vi "FlexMag - 24-03-2023.vi"() -> ()   [LabVIEW 2018] (continued)
                                n18129 = local read "abort ch1"() -> (w22192:bool)
                                n18130 = Wait Until Next ms Multiple(millisecond multiple=u32 200) -> ()  [unwired: 1 out]
                                n18131 = Not(x=w22194) -> (.not. x?=w22193:bool)
                                n18132 = Compound Arithmetic op=OR(w22190, w22192, w22193) -> (w22191:bool)
                                }
                              }
                            }
                          }
                        }
                      }
                      frame True {
                      }
                    }
                  }
                }
              }
              frame #16 {
                n18133 = local read "ch1 shutdown alg"() -> (w22200:bool)
                n18134 = case shown="True" w22200 {
                  frame False {
                  }
                  frame True {
                    n18135 = local read "abort ch1"() -> (w22201:bool)
                    n18136 = case shown="False" w22201 {
                      frame False {
                        n18137 = local read "ch1 vent?"() -> (w22202:bool)
                        n18138 = case shown="False" w22202 {
                          frame False {
                            n18139 = local write "ch1 sd pcgv close led"(TRUE ("ch1 sd cc close led")) -> ()
                            n18140 = Wait (ms)(milliseconds to wait=u32 1000) -> ()  [unwired: 1 out]
                          }
                          frame True {
                            n18141 = local write "ch1 sd pcgv open led"(TRUE ("ch1 sd cc close led")) -> ()
                            n18142 = Wait (ms)(milliseconds to wait=u32 1000) -> ()  [unwired: 1 out]
                          }
                        }
                      }
                      frame True {
                      }
                    }
                  }
                }
              }
              frame #17 {
                n18143 = local read "ch1 shutdown alg"() -> (w22207:bool)
                n18144 = case shown="True" w22207 {
                  frame False {
                  }
                  frame True {
                    n18145 = local read "abort ch1"() -> (w22208:bool)
                    n18146 = case shown="False" w22208 {
                      frame False {
                        n18147 = local read "ch1 vent?"() -> (w22209:bool)
                        n18148 = case shown="True" w22209 {
                          frame False {
                            n18149 = while {
                              i -> [w22216]
                              stop <- w22212 stop-if-true
                              n18150 = Greater Or Equal?(x=w22216, y=200) -> (x >= y?=w22218:bool)
                              n18151 = case shown="True" w22218 {
                                frame False {
                                }
                                frame True {
                                n18152 = local write "ch1 shutdown error"(TRUE ("ch1 pumpdown error")) -> ()
                                n18153 = local write "Warning Message"("CH1 ShutDown process  is canceled !\nCH1 Trns BP Left couldn't be closed" ("Warning Message")) -> ()
                                }
                              }
                              n18154 = local read "CH1_Trns_BP_Left_DI"() -> (w22211:bool)
                              n18155 = case shown="True" w22211 {
                                tunnel: [TRUE FALSE] -> w22210
                                frame False {
                                }
                                frame True {
                                n18156 = Wait Until Next ms Multiple(millisecond multiple=u32 200) -> ()  [unwired: 1 out]
                                n18157 = local write "CH1_Trns_BP_Left_DO"(FALSE ("CH1_WFC_DO")) -> ()
                                }
                              }
                              n18158 = local read "abort ch1"() -> (w22213:bool)
                              n18159 = local read "ch1 shutdown alg"() -> (w22215:bool)
                              n18160 = Not(x=w22215) -> (.not. x?=w22214:bool)
                              n18161 = Compound Arithmetic op=OR(w22210, w22213, w22214) -> (w22212:bool)
                            }
                          }
                          frame True {
                            n18162 = local read "ch1_2 vacuum level"() -> (w22226:string)
                            n18163 = Equal?(x=w22226, y="VACUUM") -> (x = y?=w22227:bool)
                            n18164 = case shown="True" w22227 {
                              frame False {
                              }
                              frame True {
                                n18165 = while {
                                i -> [w22234]
                                stop <- w22230 stop-if-true
                                n18166 = Greater Or Equal?(x=w22234, y=100) -> (x >= y?=w22236:bool)
                                n18167 = case shown="True" w22236 {
                                frame False {
                                }
                                frame True {
                                n18168 = local write "ch1 shutdown error"(TRUE ("ch1 pumpdown error")) -> ()
                                n18169 = local write "Warning Message"("CH1 ShutDown process  is canceled !\nCH1 Trns BP Left couldn't be opened" ("Warning Message")) -> ()
                                }
                                }
                                n18170 = local read "CH1_Trns_BP_Left_DI"() -> (w22229:bool)
                                n18171 = case shown="False" w22229 {
                                tunnel: [FALSE TRUE] -> w22228
                                frame False {
                                n18172 = Wait Until Next ms Multiple(millisecond multiple=u32 200) -> ()  [unwired: 1 out]
                                n18173 = local write "CH1_Trns_BP_Left_DO"(TRUE ("CH1_WFC_DO")) -> ()
                                }
                                frame True {
                                }
                                }
                                n18174 = local read "ch1 shutdown alg"() -> (w22233:bool)
                                n18175 = local read "abort ch1"() -> (w22231:bool)
                                n18176 = Not(x=w22233) -> (.not. x?=w22232:bool)
                                n18177 = Compound Arithmetic op=OR(w22228, w22231, w22232) -> (w22230:bool)
                                }
                              }
                            }
                          }
                        }
                      }
                      frame True {
                      }
                    }
                  }
                }
              }
              frame #18 {
                n18178 = local read "ch1 shutdown alg"() -> (w22243:bool)
                n18179 = case shown="True" w22243 {
                  frame False {
                  }
                  frame True {
                    n18180 = local read "abort ch1"() -> (w22244:bool)
                    n18181 = case shown="False" w22244 {
                      frame False {
                        n18182 = local read "ch1 vent?"() -> (w22245:bool)
                        n18183 = case shown="False" w22245 {
                          frame False {
                            n18184 = local write "ch1 sd trns bp left close led"(TRUE ("ch1 sd cc close led")) -> ()
                            n18185 = Wait (ms)(milliseconds to wait=u32 1000) -> ()  [unwired: 1 out]
                          }
                          frame True {
                            n18186 = local write "ch1 sd trns bp left open led"(TRUE ("ch1 sd cc close led")) -> ()
                            n18187 = Wait (ms)(milliseconds to wait=u32 1000) -> ()  [unwired: 1 out]
                          }
                        }
                      }
                      frame True {
                      }
                    }
                  }
                }
              }
              frame #19 {
                n18188 = local read "ch1 shutdown alg"() -> (w22250:bool)
                n18189 = case shown="True" w22250 {
                  frame False {
                  }
                  frame True {
                    n18190 = local read "abort ch1"() -> (w22251:bool)
                    n18191 = case shown="False" w22251 {
                      frame False {
                        n18192 = local read "ch1 vent?"() -> (w22252:bool)
                        n18193 = case shown="True" w22252 {
                          frame False {
                          }
                          frame True {
                            n18194 = while {
                              i -> [w22255]
                              stop <- w22258 stop-if-true
                              n18195 = Greater?(x=w22255, y=100) -> (0:w22254:bool)
                              n18196 = case shown="True" w22254 {
                                frame False {
                                }
                                frame True {
                                n18197 = local write "Warning Message"("CH1 ShutDown process  is canceled !\nCH1 CH VBV couldn't be opened" ("Warning Message")) -> ()
                                n18198 = local write "ch1 shutdown error"(TRUE ("ch1 pumpdown error")) -> ()
                                }
                              }
                              n18199 = local read "CH1_CH_VBV_DI"() -> (w22253:bool)
                              n18200 = case shown="False" w22253 {
                                tunnel: [FALSE TRUE] -> w22257
                                frame False {
                                n18201 = Wait Until Next ms Multiple(millisecond multiple=u32 200) -> ()  [unwired: 1 out]
                                n18202 = local write "CH1_CH_VBV_DO"(TRUE ("CH1_WFC_DO")) -> ()
                                }
                                frame True {
                                }
                              }
                              n18203 = local read "ch1 shutdown alg"() -> (w22259:bool)
                              n18204 = local read "abort ch1"() -> (w22261:bool)
                              n18205 = Not(x=w22259) -> (.not. x?=w22260:bool)
                              n18206 = Compound Arithmetic op=OR(w22257, w22261, w22260) -> (w22258:bool)
                            }
                          }
                        }
                      }
                      frame True {
                      }
                    }
                  }
                }
              }
              frame #20 {
                n18207 = local read "ch1 shutdown alg"() -> (w22268:bool)
                n18208 = case shown="True" w22268 {
                  frame False {
                  }
                  frame True {
                    n18209 = local read "abort ch1"() -> (w22269:bool)
                    n18210 = case shown="False" w22269 {
                      frame False {
                        n18211 = local read "ch1 vent?"() -> (w22270:bool)
                        n18212 = case shown="True" w22270 {
                          frame False {
                          }
                          frame True {
                            n18213 = local write "ch1 sd ch vbv open led"(TRUE ("ch1 sd cc close led")) -> ()
                            n18214 = Wait (ms)(milliseconds to wait=u32 1000) -> ()  [unwired: 1 out]
                          }
                        }
                      }
                      frame True {
                      }
                    }
                  }
                }
              }
              frame #21 {
                n18215 = local read "ch1 shutdown alg"() -> (w22273:bool)
                n18216 = case shown="True" w22273 {
                  frame False {
                  }
                  frame True {
                    n18217 = local read "abort ch1"() -> (w22274:bool)
                    n18218 = case shown="False" w22274 {
                      frame False {
                        n18219 = local read "ch1 vent?"() -> (w22275:bool)
                        n18220 = case shown="True" w22275 {
                          frame False {
                            n18221 = while {
                              i -> [w22282]
                              stop <- w22278 stop-if-true
                              # "10min"
                              n18222 = Greater Or Equal?(x=w22282, y=3000) -> (x >= y?=w22284:bool)
                              n18223 = case shown="True" w22284 {
                                frame False {
                                }
                                frame True {
                                n18224 = local write "ch1 shutdown error"(TRUE ("ch1 pumpdown error")) -> ()
                                n18225 = local write "Warning Message"("CH1 ShutDown process  is canceled !\nCH1 PL ATM switch  couldn't be opened" ("Warning Message")) -> ()
                                }
                              }
                              n18226 = local read "CH1_PL_ATM_DI"() -> (w22276:bool)
                              n18227 = local read "abort ch1"() -> (w22279:bool)
                              n18228 = local read "ch1 shutdown alg"() -> (w22281:bool)
                              n18229 = case shown="False" w22276 {
                                tunnel: [FALSE TRUE] -> w22277
                                frame False {
                                n18230 = Wait Until Next ms Multiple(millisecond multiple=u32 200) -> ()  [unwired: 1 out]
                                }
                                frame True {
                                }
                              }
                              n18231 = Not(x=w22281) -> (.not. x?=w22280:bool)
                              n18232 = Compound Arithmetic op=OR(w22277, w22279, w22280) -> (w22278:bool)
                            }
                          }
                          frame True {
                            n18233 = while {
                              i -> [w22298]
                              stop <- w22294 stop-if-true
                              # "10min"
                              n18234 = Greater Or Equal?(x=w22298, y=3000) -> (x >= y?=w22300:bool)
                              n18235 = case shown="True" w22300 {
                                frame False {
                                }
                                frame True {
                                n18236 = local write "ch1 shutdown error"(TRUE ("ch1 pumpdown error")) -> ()
                                n18237 = local write "Warning Message"("CH1 ShutDown process  is canceled !\nCH1 ATM switches  couldn't be opened" ("Warning Message")) -> ()
                                }
                              }
                              n18238 = local read "CH1_CH_ATM_DI"() -> (w22292:bool)
                              n18239 = local read "CH1_PL_ATM_DI"() -> (w22291:bool)
                              n18240 = And(x=w22292, y=w22291) -> (x .and. y?=w22290:bool)
                              n18241 = local read "abort ch1"() -> (w22295:bool)
                              n18242 = local read "ch1 shutdown alg"() -> (w22297:bool)
                              n18243 = case shown="False" w22290 {
                                tunnel: [FALSE TRUE] -> w22293
                                frame False {
                                n18244 = Wait Until Next ms Multiple(millisecond multiple=u32 200) -> ()  [unwired: 1 out]
                                }
                                frame True {
                                }
                              }
                              n18245 = Not(x=w22297) -> (.not. x?=w22296:bool)
                              n18246 = Compound Arithmetic op=OR(w22293, w22295, w22296) -> (w22294:bool)
                            }
                          }
                        }
                      }
                      frame True {
                      }
                    }
                  }
                }
              }
              frame #22 {
                n18247 = local read "ch1 shutdown alg"() -> (w22306:bool)
                n18248 = case shown="True" w22306 {
                  frame False {
                  }
                  frame True {
                    n18249 = local read "abort ch1"() -> (w22307:bool)
                    n18250 = case shown="False" w22307 {
                      frame False {
                        n18251 = local read "ch1 vent?"() -> (w22308:bool)
                        n18252 = case shown="True" w22308 {
                          frame False {
                            n18253 = local write "ch1 sd PL atm on led"(TRUE ("ch1 sd cc close led")) -> ()
                            n18254 = Wait (ms)(milliseconds to wait=u32 1000) -> ()  [unwired: 1 out]
                          }
                          frame True {
                            n18255 = local write "pcgv1 auto close"(TRUE ("ch1 sd cc close led")) -> ()
                            n18256 = local write "ch1 sd PL-CH atm on led"(TRUE ("ch1 sd cc close led")) -> ()
                            n18257 = local write "CH1_Trns_BP_Left_DO"(FALSE ("ch1 sd cc close led")) -> ()
                            n18258 = Wait (ms)(milliseconds to wait=u32 500) -> ()  [unwired: 1 out]
                            n18259 = local write "ch1_2 vacuum level"("ATMOSPHERE" ("ch3_4 vacuum level")) -> ()
                          }
                        }
                      }
                      frame True {
                      }
                    }
                  }
                }
              }
              frame #23 {
                n18260 = local read "ch1 shutdown alg"() -> (w22316:bool)
                n18261 = case shown="True" w22316 {
                  frame False {
                  }
                  frame True {
                    n18262 = local read "abort ch1"() -> (w22317:bool)
                    n18263 = case shown="False" w22317 {
                      frame False {
                        n18264 = local read "ch1 vent?"() -> (w22318:bool)
                        n18265 = case shown="True" w22318 {
                          frame False {
                            w22321 = TRUE ("Buzzer DO")
                            n18266 = local write "Buzzer DO"(w22321) -> ()
                            n18267 = local write "ch1 sd completed led"(w22321) -> ()
                            n18268 = Wait (ms)(milliseconds to wait=u32 3000) -> ()  [unwired: 1 out]
                            n18269 = local write "System Status"("CH1 SHUTDOWN PROCESS COMPLETED" ("System Status")) -> ()
                          }
                          frame True {
                            w22322 = TRUE ("Buzzer DO")
                            n18270 = local write "Buzzer DO"(w22322) -> ()
                            n18271 = local write "ch1 sd completed led"(w22322) -> ()
                            n18272 = Wait (ms)(milliseconds to wait=u32 3000) -> ()  [unwired: 1 out]
                            n18273 = local write "System Status"("CH1 VENT PROCESS COMPLETED" ("System Status")) -> ()
                          }
                        }
                      }
                      frame True {
                      }
                    }
                  }
                }
              }
              frame #24 {
                n18274 = local read "ch1 shutdown alg"() -> (w22325:bool)
                n18275 = case shown="True" w22325 {
                  frame False {
                  }
                  frame True {
                    n18276 = local read "abort ch1"() -> (w22326:bool)
                    n18277 = case shown="False" w22326 {
                      frame False {
                        w22328 = FALSE ("Buzzer DO")
                        n18278 = local write "Buzzer DO"(w22328) -> ()
                        n18279 = local write "ch1 shutdown alg"(w22328) -> ()
                        n18280 = local write "Shut Down CH1"(w22328) -> ()
                        n18281 = Wait (ms)(milliseconds to wait=u32 3000) -> ()  [unwired: 1 out]
                        n18282 = local write "System Status"("SEMI-AUTOMATIC MODE " ("System Status")) -> ()
                      }
                      frame True {
                      }
                    }
                  }
                }
              }
            }
          }
          frame True {
          }
        }
      }
    }
  }
  n18283 = disable-structure shown="Disabled" {
    frame Disabled {
      n18284 = Multiply(x=u32 1000 ("millisecond multiple")) -> ()  [unwired: 1 in, 1 out]
    }
    frame Enabled {
    }
  }
  n18285 = while {
    stop <- FALSE stop-if-true
    n18286 = Wait Until Next ms Multiple(millisecond multiple=u32 300) -> ()  [unwired: 1 out]
    n18287 = Build Array(FALSE ("CH4_SRV1_Piston_For_DO"), "deactivate all trns sensors", "activate all trns sensors") -> (w22804:bool[])
    n18288 = Boolean Array To Number(Boolean array=w22804) -> (number=w22806:u32)
    n18289 = Mantissa & Exponent(0:w22806) -> (2:w22805:dbl)  [unwired: 1 out]
    n18290 = case shown="1" w22805 {
      frame 0, Default {
      }
      frame 1 {
        w22812 = TRUE ("CH4_SRV1_Piston_For_DO")
        n18291 = Wait (ms)(milliseconds to wait=u32 300) -> ()  [unwired: 1 out]
        n18292 = local write "deactivate all trns sensors"(FALSE ("deactivate all trns sensors")) -> ()
        n18293 = local write "CH2_Right_Limit_DO"(w22812) -> ()
        n18294 = local write "CH2_Right_Slow_DO"(w22812) -> ()
        n18295 = local write "CH2_Left_Slow_DO"(w22812) -> ()
        n18296 = local write "CH2_Left_Limit_DO"(w22812) -> ()
        n18297 = local write "CH3_Right_Limit_DO"(w22812) -> ()
        n18298 = local write "CH3_Right_Slow_DO"(w22812) -> ()
        n18299 = local write "CH3_Left_Slow_DO"(w22812) -> ()
        n18300 = local write "CH3_Left_Limit_DO"(w22812) -> ()
        n18301 = local write "CH4_Left_Limit_DO"(w22812) -> ()
        n18302 = local write "CH4_Left_Slow_DO"(w22812) -> ()
        n18303 = local write "CH1_Right_Limit_DO"(w22812) -> ()
        n18304 = local write "CH1_Right_Slow_DO"(w22812) -> ()
        n18305 = local write "trns sensors led"(TRUE ("trns sensors led")) -> ()
      }
      frame 2 {
        w22816 = FALSE ("CH4_SRV1_Piston_For_DO")
        n18306 = Wait (ms)(milliseconds to wait=u32 300) -> ()  [unwired: 1 out]
        n18307 = local write "activate all trns sensors"(FALSE ("activate all trns sensors")) -> ()
        n18308 = local write "CH1_Right_Limit_DO"(w22816) -> ()
        n18309 = local write "CH1_Right_Slow_DO"(w22816) -> ()
        n18310 = local write "CH2_Right_Limit_DO"(w22816) -> ()
        n18311 = local write "CH2_Right_Slow_DO"(w22816) -> ()
        n18312 = local write "CH2_Left_Slow_DO"(w22816) -> ()
        n18313 = local write "CH2_Left_Limit_DO"(w22816) -> ()
        n18314 = local write "CH3_Right_Limit_DO"(w22816) -> ()
        n18315 = local write "CH3_Right_Slow_DO"(w22816) -> ()
        n18316 = local write "CH3_Left_Slow_DO"(w22816) -> ()
        n18317 = local write "CH3_Left_Limit_DO"(w22816) -> ()
        n18318 = local write "CH4_Left_Limit_DO"(w22816) -> ()
        n18319 = local write "CH4_Left_Slow_DO"(w22816) -> ()
        n18320 = local write "trns sensors led"(FALSE ("trns sensors led")) -> ()
      }
    }
  }
  n18321 = while {
    stop <- FALSE stop-if-true
    n18322 = local read "cassette position selection"() -> (w22817:u16)
    n18323 = Build Array(FALSE, "forward roll", "back roll", "position") -> (w22819:bool[])
    n18324 = Wait Until Next ms Multiple(millisecond multiple=u32 300) -> ()  [unwired: 1 out]
    n18325 = Boolean Array To Number(Boolean array=w22819) -> (number=w22824:u32)
    n18326 = Mantissa & Exponent(0:w22824) -> (2:w22818:dbl)  [unwired: 1 out]
    n18327 = case shown="1" w22818 {
      tunnel: w22817 -> [_ w22827 w23093 w23355]
      frame 0, Default {
      }
      frame 1 {
        # "forward roll"
        n18328 = stacked-sequence {
          tunnel: w22827 -> [w22829 _ _ _ _ _ w22887 w22897 _]
          frame #0 {
            n18329 = Wait (ms)(milliseconds to wait=u32 100) -> ()  [unwired: 1 out]
            n18330 = case shown="0, Default" w22829 {
              frame 0, Default {
                n18331 = local write "roll error"(TRUE ("roll error")) -> ()
                n18332 = Wait (ms)(milliseconds to wait=u32 100) -> ()  [unwired: 1 out]
                n18333 = local write "Warning Message"("Choose Cassette Position !" ("Warning Message")) -> ()
              }
              frame 1 {
                n18334 = local read "CH1_SRV1_Piston_For_DI"() -> (w22833:bool)
                n18335 = case shown="False" w22833 {
                  frame False {
                    n18336 = local write "roll error"(TRUE ("roll error")) -> ()
                    n18337 = Wait (ms)(milliseconds to wait=u32 100) -> ()  [unwired: 1 out]
                  }
                  frame True {
                  }
                }
              }
              frame 2 {
                n18338 = local read "CH2_SRV1_Piston_For_DI"() -> (w22836:bool)
                n18339 = case shown="False" w22836 {
                  frame False {
                    n18340 = local write "roll error"(TRUE ("roll error")) -> ()
                    n18341 = Wait (ms)(milliseconds to wait=u32 100) -> ()  [unwired: 1 out]
                  }
                  frame True {
                  }
                }
              }
              frame 3 {
                n18342 = local read "CH3_SRV1_Piston_For_DI"() -> (w22839:bool)
                n18343 = case shown="False" w22839 {
                  frame False {
                    n18344 = local write "roll error"(TRUE ("roll error")) -> ()
                    n18345 = Wait (ms)(milliseconds to wait=u32 100) -> ()  [unwired: 1 out]
                  }
                  frame True {
                  }
                }
              }
              frame 4 {
                n18346 = local read "CH4_SRV1_Piston_For_DI"() -> (w22842:bool)
                n18347 = case shown="False" w22842 {
                  frame False {
                    n18348 = local write "roll error"(TRUE ("roll error")) -> ()
                    n18349 = Wait (ms)(milliseconds to wait=u32 100) -> ()  [unwired: 1 out]
                  }
                  frame True {
                  }
                }
              }
            }
          }
          frame #1 {
            n18350 = local read "forward roll"() -> (w22846:bool)
            n18351 = case shown="True" w22846 {
              frame False {
              }
              frame True {
                n18352 = flat-sequence {
                  frame #0 {
                    n18353 = local write "Roll Forw"(TRUE ("Roll Forw")) -> ()
                  }
                  frame #1 {
                    n18354 = Wait (ms)(milliseconds to wait=u32 300) -> ()  [unwired: 1 out]
                  }
                  frame #2 {
                    n18355 = local write "TC parameter set"(TRUE ("TC parameter set")) -> ()
                  }
                  frame #3 {
                    n18356 = Wait (ms)(milliseconds to wait=u32 300) -> ()  [unwired: 1 out]
                  }
                }
                n18357 = local write "lap number right actual"(0.0 ("lap number right actual")) -> ()
                n18358 = local write "lap number left actual"(0.0 ("lap number right actual")) -> ()
              }
            }
            n18359 = local read "step count"() -> (w22845:dbl)
            n18360 = local write "step count 2"(w22845) -> ()
          }
          frame #2 {
            n18361 = local read "forward roll"() -> (w22853:bool)
            n18362 = case shown="True" w22853 {
              frame False {
              }
              frame True {
                n18363 = while {
                  i -> [w22859]
                  stop <- w22857 stop-if-true
                  n18364 = Wait Until Next ms Multiple(millisecond multiple=u32 300) -> ()  [unwired: 1 out]
                  n18365 = local read "TC parameter set"() -> (w22863:bool)
                  n18366 = local read "forward roll"() -> (w22855:bool)
                  n18367 = local read "ABORT"() -> (w22861:bool)
                  n18368 = Not(x=w22863) -> (.not. x?=w22860:bool)
                  n18369 = Not(x=w22855) -> (.not. x?=w22854:bool)
                  n18370 = Greater Or Equal?(x=w22859, y=u32 400 ("millisecond multiple")) -> (x >= y?=w22856:bool)
                  n18371 = Compound Arithmetic op=OR(w22856, w22860, w22861, w22854) -> (w22857:bool)
                  n18372 = local write "roll error"(w22856) -> ()
                }
              }
            }
          }
          frame #3 {
            n18373 = local read "forward roll"() -> (w22864:bool)
            n18374 = case shown="True" w22864 {
              frame False {
              }
              frame True {
                n18375 = flat-sequence {
                  frame #0 {
                    n18376 = disable-structure shown="Enabled" {
                      disable-tunnel: [w22868 0.1 ("current voltage")] -> w22865
                      frame Disabled {
                        n18377 = local read "output_pid"() -> (w22868:dbl)
                      }
                      frame Enabled {
                      }
                    }
                    n18378 = local read "tension value"() -> (w22867:dbl)
                    n18379 = local write "TC1_set_value"(w22867) -> ()
                    n18380 = local write "TC2_overspeed_value"(w22865) -> ()
                    n18381 = local write "current voltage"(w22865) -> ()
                    n18382 = Wait (ms)(milliseconds to wait=u32 1000) -> ()  [unwired: 1 out]
                  }
                  frame #1 {
                    n18383 = local write "TC2_overspeed_set"(TRUE ("TC2 Set moxa")) -> ()
                    n18384 = local write "TC1_auto_set"(TRUE ("TC1_set")) -> ()
                  }
                  frame #2 {
                    n18385 = local write "TC1_overspeed_value"(sgl 0.0 ("TC2_set_value")) -> ()
                    n18386 = local write "TC2_set_value"(sgl 0.0 ("TC2_set_value")) -> ()
                    n18387 = Wait (ms)(milliseconds to wait=u32 2000) -> ()  [unwired: 1 out]
                  }
                  frame #3 {
                    n18388 = local write "TC1_overspeed_set"(TRUE ("TC2_auto_set")) -> ()
                    n18389 = local write "TC2_auto_set"(TRUE ("TC2_auto_set")) -> ()
                  }
                }
              }
            }
          }
          frame #4 {
            n18390 = local read "forward roll"() -> (w22877:bool)
            n18391 = case shown="True" w22877 {
              frame False {
              }
              frame True {
                n18392 = flat-sequence {
                  frame #0 {
                    w22879 = TRUE ("CH1_SRV_Direction_Clockwise_DO")
                    n18393 = disable-structure shown="Disabled" {
                      frame Disabled {
                        n18394 = local write "setpoint"(0.1 ("setpoint")) -> ()
                      }
                      frame Enabled {
                      }
                    }
                    n18395 = local write "CH1_SRV_Direction_Clockwise_DO"(w22879) -> ()
                    n18396 = local write "CH2_SRV_Direction_Clockwise_DO"(w22879) -> ()
                    n18397 = local write "CH3_SRV_Direction_Clockwise_DO"(w22879) -> ()
                    n18398 = local write "CH4_SRV_Direction_Clockwise_DO"(w22879) -> ()
                    n18399 = Wait (ms)(milliseconds to wait=u32 100) -> ()  [unwired: 1 out]
                  }
                  frame #1 {
                    n18400 = Wait (ms)(milliseconds to wait=u32 3000) -> ()  [unwired: 1 out]
                  }
                }
              }
            }
          }
          frame #5 {
            n18401 = local read "forward roll"() -> (w22882:bool)
            n18402 = case shown="True" w22882 {
              frame False {
              }
              frame True {
                n18403 = Wait (ms)(milliseconds to wait=u32 100) -> ()  [unwired: 1 out]
                n18404 = local write "Tension_Controllers_Start/Stop DO"(TRUE ("CH1_SRV_Direction_Clockwise_DO")) -> ()
                n18405 = disable-structure shown="Disabled" {
                  frame Disabled {
                    w22885 = 0.1 ("lower limit")
                    n18406 = Bundle("lower limit"=w22885, "lower limit"=w22885) -> (w22886:cluster{"lower limit":dbl, "lower limit":dbl})  [unwired: 1 in]
                    n18407 = local write "output range"(w22886) -> ()
                  }
                  frame Enabled {
                  }
                }
              }
            }
          }
          frame #6 {
            n18408 = local read "forward roll"() -> (w22888:bool)
            n18409 = case shown="True" w22888 {
              tunnel: w22887 -> [_ w22891]
              frame False {
              }
              frame True {
                n18410 = case shown="3" w22891 {
                  frame 0, Default {
                    n18411 = local write "roll error"(TRUE ("roll error")) -> ()
                  }
                  frame 1 {
                    n18412 = local write "CH1_Motor DO"(TRUE ("CH1_Motor DO")) -> ()
                  }
                  frame 2 {
                    n18413 = local write "CH2_Motor DO"(TRUE ("CH1_Motor DO")) -> ()
                  }
                  frame 3 {
                    n18414 = local write "CH3_Motor DO"(TRUE ("CH1_Motor DO")) -> ()
                  }
                  frame 4 {
                    n18415 = local write "CH4_Motor DO"(TRUE ("CH1_Motor DO")) -> ()
                  }
                }
                n18416 = local write "QR continuous mode"(TRUE ("QR continuous mode")) -> ()
                n18417 = local write "pid output"(TRUE ("pid output")) -> ()
              }
            }
          }
          frame #7 {
            n18418 = local read "forward roll"() -> (w22898:bool)
            n18419 = case shown="True" w22898 {
              tunnel: w22897 -> [_ w22899]
              frame False {
              }
              frame True {
                n18420 = case shown="1" w22899 {
                  frame 0, Default {
                    n18421 = local write "roll error"(TRUE ("roll error")) -> ()
                  }
                  frame 1 {
                    n18422 = while {
                      i -> [w22924]
                      stop <- w22932 stop-if-true
                      n18423 = local read "CH1_SRV2_COUNTER_DI"() -> (w22928:bool)
                      n18424 = local read "Ch1_srv1_counter DI"() -> (w22919:bool)
                      n18425 = feedback #322() -> (w22929:bool)  [unwired: 1 in]
                      n18426 = feedback-in #322(w22928) -> ()
                      n18427 = feedback #323() -> (w22918:bool)  [unwired: 1 in]
                      n18428 = feedback-in #323(w22919) -> ()
                      n18429 = Implies(1:w22928, 2:w22929) -> (0:w22930:bool)
                      n18430 = Not(x=w22930) -> (.not. x?=w22927:bool)
                      n18431 = Greater Or Equal?(x=w22924, y=200) -> (x >= y?=w22920:bool)
                      n18432 = Implies(1:w22919, 2:w22918) -> (0:w22917:bool)
                      n18433 = case shown="True" w22927 {
                        frame False {
                        }
                        frame True {
                          n18434 = local read "output range"() -> (w22940:cluster{"output high":dbl, "output low":dbl})
                          n18435 = local read "lap number right actual"() -> (w22947:dbl)
                          n18436 = Unbundle By Name(w22940) -> ("output high"=w22942:dbl, "output low"=w22945:dbl)
                          n18437 = local read "decreasing voltage"() -> (w22941:dbl)
                          n18438 = Increment(x=w22947) -> (x+1=w22946:dbl)
                          n18439 = local write "lap number right actual"(w22946) -> ()
                          n18440 = Subtract(x=w22942, y=w22941) -> (x-y=w22944:dbl)
                          n18441 = Bundle(w22944, "output low"=w22945) -> (w22943:cluster{dbl, "output low":dbl})  [unwired: 1 in]
                          n18442 = local write "output range"(w22943) -> ()
                        }
                      }
                      n18443 = Not(x=w22917) -> (.not. x?=w22916:bool)
                      n18444 = case shown="True" w22916 {
                        frame False {
                        }
                        frame True {
                          n18445 = local read "lap number left actual"() -> (w22937:dbl)
                          n18446 = Increment(x=w22937) -> (x+1=w22936:dbl)
                          n18447 = local write "lap number left actual"(w22936) -> ()
                        }
                      }
                      n18448 = case shown="True" w22920 {
                        tunnel: [FALSE w22939] -> w22925
                        frame False {
                        }
                        frame True {
                          n18449 = local read "forroll stop cmd"() -> (w22939:bool)
                        }
                      }
                      n18450 = local read "lap number right actual"() -> (w22922:dbl)
                      n18451 = local read "max rotation number"() -> (w22923:dbl)
                      n18452 = local read "lap number left actual"() -> (w22915:dbl)
                      n18453 = local read "max rotation number"() -> (w22914:dbl)
                      n18454 = Greater Or Equal?(x=w22915, y=w22914) -> (x >= y?=w22913:bool)
                      n18455 = Greater Or Equal?(x=w22922, y=w22923) -> (x >= y?=w22912:bool)
                      n18456 = local read "abort ch1"() -> (w22926:bool)
                      n18457 = local read "forward roll"() -> (w22935:bool)
                      n18458 = Or(x=w22913, y=w22912) -> (x .or. y?=w22911:bool)
                      n18459 = Not(x=w22935) -> (.not. x?=w22934:bool)
                      n18460 = Compound Arithmetic op=OR(w22926, w22934, w22925, w22911) -> (w22932:bool)
                      n18461 = Not(x=w22932) -> (.not. x?=w22933:bool)
                      n18462 = local write "CH1_Motor DO"(w22933) -> ()
                      n18463 = Wait Until Next ms Multiple(millisecond multiple=u32 100) -> ()  [unwired: 1 out]
                    }
                    n18464 = while {
                      stop <- w22907 stop-if-true
                      n18465 = stacked-sequence {
                        frame #0 {
                          n18466 = local read "output_pid"() -> (w22908:dbl)
                          n18467 = Wait (ms)(milliseconds to wait=u32 25) -> ()  [unwired: 1 out]
                          n18468 = local write "TC2_overspeed_value"(w22908) -> ()
                          n18469 = local write "current voltage"(w22908) -> ()
                        }
                        frame #1 {
                          n18470 = local write "TC2_overspeed_set"(TRUE ("TC2_overspeed_set")) -> ()
                        }
                      }
                      n18471 = local read "CH1_Motor DO"() -> (w22902:bool)
                      n18472 = local read "forward roll"() -> (w22905:bool)
                      n18473 = local read "abort ch1"() -> (w22906:bool)
                      n18474 = local read "set speed (ms)"() -> (w22903:u32)
                      n18475 = Not(x=w22902) -> (.not. x?=w22901:bool)
                      n18476 = Not(x=w22905) -> (.not. x?=w22904:bool)
                      n18477 = Compound Arithmetic op=OR(w22901, w22906, w22904) -> (w22907:bool)
                      n18478 = Wait Until Next ms Multiple(millisecond multiple=w22903) -> ()  [unwired: 1 out]
                    }
                  }
                  frame 2 {
                    n18479 = while {
                      i -> [w22971]
                      stop <- w22979 stop-if-true
                      n18480 = local read "CH2_SRV2_COUNTER_DI"() -> (w22975:bool)
                      n18481 = local read "Ch2_srv1_counter DI"() -> (w22968:bool)
                      n18482 = Greater Or Equal?(x=w22971, y=200) -> (x >= y?=w22963:bool)
                      n18483 = case shown="True" w22963 {
                        tunnel: [FALSE w22984] -> w22972
                        frame False {
                        }
                        frame True {
                          n18484 = local read "forroll stop cmd"() -> (w22984:bool)
                        }
                      }
                      n18485 = feedback #324() -> (w22976:bool)  [unwired: 1 in]
                      n18486 = feedback-in #324(w22975) -> ()
                      n18487 = Implies(1:w22975, 2:w22976) -> (0:w22977:bool)
                      n18488 = Not(x=w22977) -> (.not. x?=w22974:bool)
                      n18489 = feedback #325() -> (w22967:bool)  [unwired: 1 in]
                      n18490 = feedback-in #325(w22968) -> ()
                      n18491 = case shown="True" w22974 {
                        frame False {
                        }
                        frame True {
                          n18492 = local read "output range"() -> (w22992:cluster{"output high":dbl, "output low":dbl})
                          n18493 = local read "lap number right actual"() -> (w22994:dbl)
                          n18494 = Unbundle By Name(w22992) -> ("output high"=w22990:dbl, "output low"=w22987:dbl)
                          n18495 = Increment(x=w22994) -> (x+1=w22993:dbl)
                          n18496 = local write "lap number right actual"(w22993) -> ()
                          n18497 = local read "decreasing voltage"() -> (w22991:dbl)
                          n18498 = Subtract(x=w22990, y=w22991) -> (x-y=w22988:dbl)
                          n18499 = Bundle(w22988, "output low"=w22987) -> (w22989:cluster{dbl, "output low":dbl})  [unwired: 1 in]
                          n18500 = local write "output range"(w22989) -> ()
                        }
                      }
                      n18501 = Implies(1:w22968, 2:w22967) -> (0:w22966:bool)
                      n18502 = Not(x=w22966) -> (.not. x?=w22965:bool)
                      n18503 = case shown="True" w22965 {
                        frame False {
                        }
                        frame True {
                          n18504 = local read "lap number left actual"() -> (w22986:dbl)
                          n18505 = Increment(x=w22986) -> (x+1=w22985:dbl)
                          n18506 = local write "lap number left actual"(w22985) -> ()
                        }
                      }
                      n18507 = local read "lap number left actual"() -> (w22961:dbl)
                      n18508 = local read "max rotation number"() -> (w22962:dbl)
                      n18509 = local read "lap number right actual"() -> (w22970:dbl)
                      n18510 = local read "max rotation number"() -> (w22969:dbl)
                      n18511 = Greater Or Equal?(x=w22961, y=w22962) -> (x >= y?=w22960:bool)
                      n18512 = Greater Or Equal?(x=w22970, y=w22969) -> (x >= y?=w22959:bool)
                      n18513 = local read "abort ch2"() -> (w22973:bool)
                      n18514 = local read "forward roll"() -> (w22982:bool)
                      n18515 = Or(x=w22960, y=w22959) -> (x .or. y?=w22958:bool)
                      n18516 = Not(x=w22982) -> (.not. x?=w22981:bool)
                      n18517 = Compound Arithmetic op=OR(w22973, w22981, w22972, w22958) -> (w22979:bool)
                      n18518 = Not(x=w22979) -> (.not. x?=w22980:bool)
                      n18519 = local write "CH2_Motor DO"(w22980) -> ()
                      n18520 = Wait Until Next ms Multiple(millisecond multiple=u32 100) -> ()  [unwired: 1 out]
                    }
                    n18521 = while {
                      stop <- w22954 stop-if-true
                      n18522 = stacked-sequence {
                        frame #0 {
                          n18523 = local read "output_pid"() -> (w22955:dbl)
                          n18524 = Wait (ms)(milliseconds to wait=u32 25) -> ()  [unwired: 1 out]
                          n18525 = local write "TC2_overspeed_value"(w22955) -> ()
                          n18526 = local write "current voltage"(w22955) -> ()
                        }
                        frame #1 {
                          n18527 = local write "TC2_overspeed_set"(TRUE ("TC2_overspeed_set")) -> ()
                        }
                      }
                      n18528 = local read "CH2_Motor DO"() -> (w22949:bool)
                      n18529 = local read "forward roll"() -> (w22952:bool)
                      n18530 = local read "set speed (ms)"() -> (w22950:u32)
                      n18531 = local read "abort ch2"() -> (w22953:bool)
                      n18532 = Not(x=w22949) -> (.not. x?=w22948:bool)
                      n18533 = Not(x=w22952) -> (.not. x?=w22951:bool)
                      n18534 = Compound Arithmetic op=OR(w22948, w22953, w22951) -> (w22954:bool)
                      n18535 = Wait Until Next ms Multiple(millisecond multiple=w22950) -> ()  [unwired: 1 out]
                    }
                  }
                  frame 3 {
                    n18536 = while {
                      i -> [w23018]
                      stop <- w23026 stop-if-true
                      n18537 = local read "CH3_SRV2_COUNTER_DI"() -> (w23022:bool)
                      n18538 = local read "Ch3_srv1_counter DI"() -> (w23015:bool)
                      n18539 = feedback #326() -> (w23023:bool)  [unwired: 1 in]
                      n18540 = feedback-in #326(w23022) -> ()
                      n18541 = Greater Or Equal?(x=w23018, y=200) -> (x >= y?=w23010:bool)
                      n18542 = Implies(1:w23022, 2:w23023) -> (0:w23024:bool)
                      n18543 = Not(x=w23024) -> (.not. x?=w23021:bool)
                      n18544 = case shown="True" w23010 {
                        tunnel: [FALSE w23031] -> w23019
                        frame False {
                        }
                        frame True {
                          n18545 = local read "forroll stop cmd"() -> (w23031:bool)
                        }
                      }
                      n18546 = case shown="True" w23021 {
                        frame False {
                        }
                        frame True {
                          n18547 = local read "lap number right actual"() -> (w23041:dbl)
                          n18548 = local read "output range"() -> (w23034:cluster{"output high":dbl, "output low":dbl})
                          n18549 = Unbundle By Name(w23034) -> ("output high"=w23036:dbl, "output low"=w23039:dbl)
                          n18550 = Increment(x=w23041) -> (x+1=w23040:dbl)
                          n18551 = local write "lap number right actual"(w23040) -> ()
                          n18552 = local read "decreasing voltage"() -> (w23035:dbl)
                          n18553 = Subtract(x=w23036, y=w23035) -> (x-y=w23038:dbl)
                          n18554 = Bundle(w23038, "output low"=w23039) -> (w23037:cluster{dbl, "output low":dbl})  [unwired: 1 in]
                          n18555 = local write "output range"(w23037) -> ()
                        }
                      }
                      n18556 = feedback #327() -> (w23014:bool)  [unwired: 1 in]
                      n18557 = feedback-in #327(w23015) -> ()
                      n18558 = Implies(1:w23015, 2:w23014) -> (0:w23013:bool)
                      n18559 = Not(x=w23013) -> (.not. x?=w23012:bool)
                      n18560 = case shown="True" w23012 {
                        frame False {
                        }
                        frame True {
                          n18561 = local read "lap number left actual"() -> (w23033:dbl)
                          n18562 = Increment(x=w23033) -> (x+1=w23032:dbl)
                          n18563 = local write "lap number left actual"(w23032) -> ()
                        }
                      }
                      n18564 = local read "lap number right actual"() -> (w23017:dbl)
                      n18565 = local read "lap number left actual"() -> (w23009:dbl)
                      n18566 = local read "max rotation number"() -> (w23008:dbl)
                      n18567 = local read "max rotation number"() -> (w23016:dbl)
                      n18568 = local read "abort ch3"() -> (w23020:bool)
                      n18569 = local read "forward roll"() -> (w23029:bool)
                      n18570 = Greater Or Equal?(x=w23009, y=w23008) -> (x >= y?=w23006:bool)
                      n18571 = Greater Or Equal?(x=w23017, y=w23016) -> (x >= y?=w23007:bool)
                      n18572 = Or(x=w23007, y=w23006) -> (x .or. y?=w23005:bool)
                      n18573 = Not(x=w23029) -> (.not. x?=w23028:bool)
                      n18574 = Compound Arithmetic op=OR(w23020, w23028, w23019, w23005) -> (w23026:bool)
                      n18575 = Not(x=w23026) -> (.not. x?=w23027:bool)
                      n18576 = local write "CH3_Motor DO"(w23027) -> ()
                      n18577 = Wait Until Next ms Multiple(millisecond multiple=u32 100) -> ()  [unwired: 1 out]
                    }
                    n18578 = while {
                      stop <- w23001 stop-if-true
                      n18579 = stacked-sequence {
                        frame #0 {
                          n18580 = local read "output_pid"() -> (w23002:dbl)
                          n18581 = Wait (ms)(milliseconds to wait=u32 25) -> ()  [unwired: 1 out]
                          n18582 = local write "TC2_overspeed_value"(w23002) -> ()
                          n18583 = local write "current voltage"(w23002) -> ()
                        }
                        frame #1 {
                          n18584 = local write "TC2_overspeed_set"(TRUE ("TC2_overspeed_set")) -> ()
                        }
                      }
                      n18585 = local read "CH3_Motor DO"() -> (w22996:bool)
                      n18586 = local read "forward roll"() -> (w22999:bool)
                      n18587 = local read "set speed (ms)"() -> (w22997:u32)
                      n18588 = local read "abort ch3"() -> (w23000:bool)
                      n18589 = Not(x=w22996) -> (.not. x?=w22995:bool)
                      n18590 = Not(x=w22999) -> (.not. x?=w22998:bool)
                      n18591 = Compound Arithmetic op=OR(w22995, w23000, w22998) -> (w23001:bool)
                      n18592 = Wait Until Next ms Multiple(millisecond multiple=w22997) -> ()  [unwired: 1 out]
                    }
                  }
                  frame 4 {
                    n18593 = while {
                      i -> [w23064]
                      stop <- w23073 stop-if-true
                      n18594 = local read "CH4_SRV2_COUNTER_DI"() -> (w23069:bool)
                      n18595 = local read "Ch4_srv1_counter DI"() -> (w23057:bool)
                      n18596 = feedback #328() -> (w23070:bool)  [unwired: 1 in]
                      n18597 = feedback-in #328(w23069) -> ()
                      n18598 = Greater Or Equal?(x=w23064, y=200) -> (x >= y?=w23065:bool)
                      n18599 = Implies(1:w23069, 2:w23070) -> (0:w23071:bool)
                      n18600 = Not(x=w23071) -> (.not. x?=w23068:bool)
                      n18601 = case shown="True" w23065 {
                        tunnel: [FALSE w23078] -> w23066
                        frame False {
                        }
                        frame True {
                          n18602 = local read "forroll stop cmd"() -> (w23078:bool)
                        }
                      }
                      n18603 = case shown="True" w23068 {
                        frame False {
                        }
                        frame True {
                          n18604 = local read "lap number right actual"() -> (w23088:dbl)
                          n18605 = local read "output range"() -> (w23086:cluster{"output high":dbl, "output low":dbl})
                          n18606 = Unbundle By Name(w23086) -> ("output high"=w23084:dbl, "output low"=w23081:dbl)
                          n18607 = Increment(x=w23088) -> (x+1=w23087:dbl)
                          n18608 = local write "lap number right actual"(w23087) -> ()
                          n18609 = local read "decreasing voltage"() -> (w23085:dbl)
                          n18610 = Subtract(x=w23084, y=w23085) -> (x-y=w23082:dbl)
                          n18611 = Bundle(w23082, "output low"=w23081) -> (w23083:cluster{dbl, "output low":dbl})  [unwired: 1 in]
                          n18612 = local write "output range"(w23083) -> ()
                        }
                      }
                      n18613 = feedback #329() -> (w23058:bool)  [unwired: 1 in]
                      n18614 = feedback-in #329(w23057) -> ()
                      n18615 = Implies(1:w23057, 2:w23058) -> (0:w23059:bool)
                      n18616 = Not(x=w23059) -> (.not. x?=w23060:bool)
                      n18617 = case shown="True" w23060 {
                        frame False {
                        }
                        frame True {
                          n18618 = local read "lap number left actual"() -> (w23080:dbl)
                          n18619 = Increment(x=w23080) -> (x+1=w23079:dbl)
                          n18620 = local write "lap number left actual"(w23079) -> ()
                        }
                      }
                      n18621 = local read "lap number right actual"() -> (w23061:dbl)
                      n18622 = local read "lap number left actual"() -> (w23056:dbl)
                      n18623 = local read "max rotation number"() -> (w23062:dbl)
                      n18624 = local read "max rotation number"() -> (w23055:dbl)
                      n18625 = local read "abort ch4"() -> (w23067:bool)
                      n18626 = local read "forward roll"() -> (w23076:bool)
                      n18627 = Greater Or Equal?(x=w23061, y=w23062) -> (x >= y?=w23053:bool)
                      n18628 = Greater Or Equal?(x=w23056, y=w23055) -> (x >= y?=w23052:bool)
                      n18629 = Not(x=w23076) -> (.not. x?=w23075:bool)
                      n18630 = Or(x=w23053, y=w23052) -> (x .or. y?=w23054:bool)
                      n18631 = Compound Arithmetic op=OR(w23067, w23075, w23066, w23054) -> (w23073:bool)
                      n18632 = Not(x=w23073) -> (.not. x?=w23074:bool)
                      n18633 = local write "CH4_Motor DO"(w23074) -> ()
                      n18634 = Wait Until Next ms Multiple(millisecond multiple=u32 100) -> ()  [unwired: 1 out]
                    }
                    n18635 = while {
                      stop <- w23048 stop-if-true
                      n18636 = stacked-sequence {
                        frame #0 {
                          n18637 = local read "output_pid"() -> (w23049:dbl)
                          n18638 = Wait (ms)(milliseconds to wait=u32 25) -> ()  [unwired: 1 out]
                          n18639 = local write "TC2_overspeed_value"(w23049) -> ()
                          n18640 = local write "current voltage"(w23049) -> ()
                        }
                        frame #1 {
                          n18641 = local write "TC2_overspeed_set"(TRUE ("TC2_overspeed_set")) -> ()
                        }
                      }
                      n18642 = local read "CH4_Motor DO"() -> (w23043:bool)
                      n18643 = local read "forward roll"() -> (w23046:bool)
                      n18644 = local read "abort ch4"() -> (w23047:bool)
                      n18645 = local read "set speed (ms)"() -> (w23044:u32)
                      n18646 = Not(x=w23043) -> (.not. x?=w23042:bool)
                      n18647 = Not(x=w23046) -> (.not. x?=w23045:bool)
                      n18648 = Compound Arithmetic op=OR(w23042, w23047, w23045) -> (w23048:bool)
                      n18649 = Wait Until Next ms Multiple(millisecond multiple=w23044) -> ()  [unwired: 1 out]
                    }
                  }
                }
              }
            }
          }
          frame #8 {
            w23090 = FALSE ("forward roll")
            n18650 = local write "Tension_Controllers_Start/Stop DO"(w23090) -> ()
            n18651 = local write "CH1_Motor DO"(w23090) -> ()